vi "TLB Native Dynamic Events ver 0.26a.vi"() -> ()   [LabVIEW 2018] (continued)
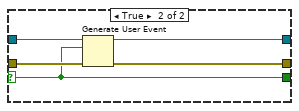
[diagram p2: hidden frame]
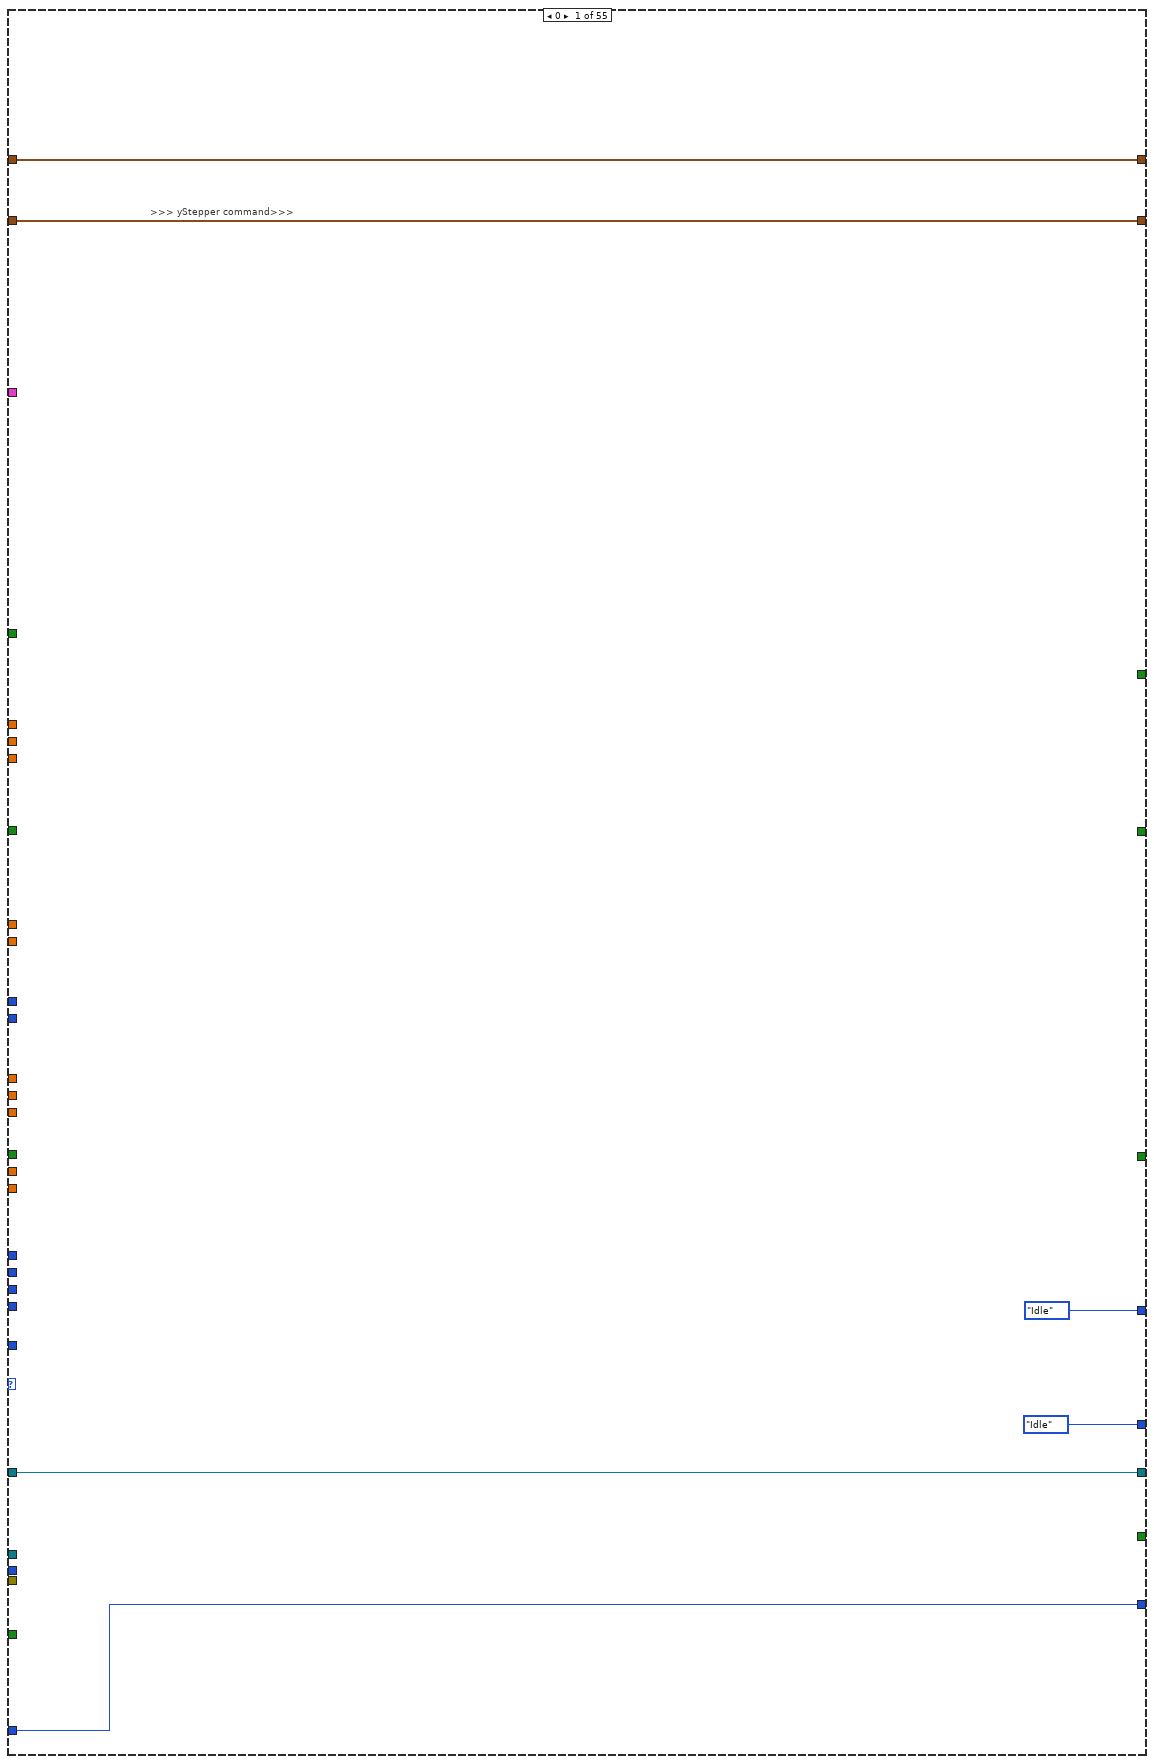
[diagram p5: hidden frame]
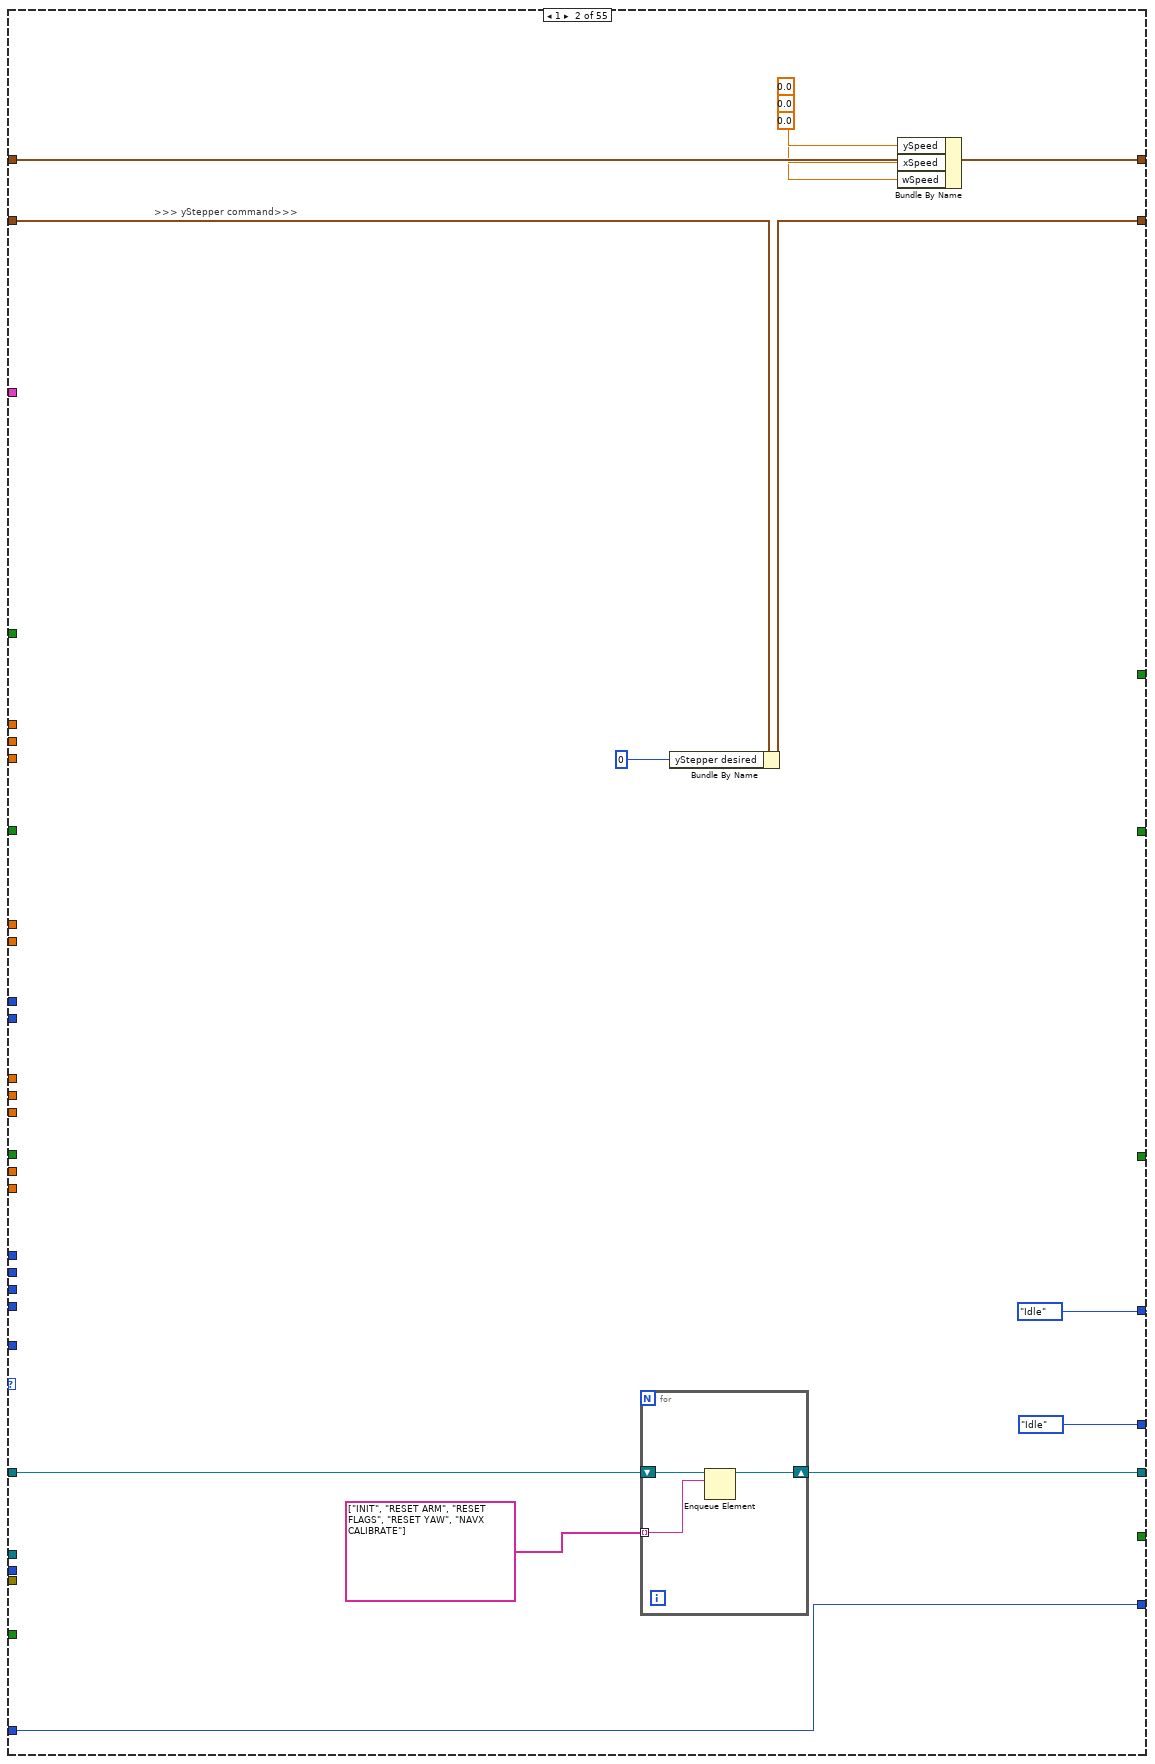
[diagram p6: hidden frame]
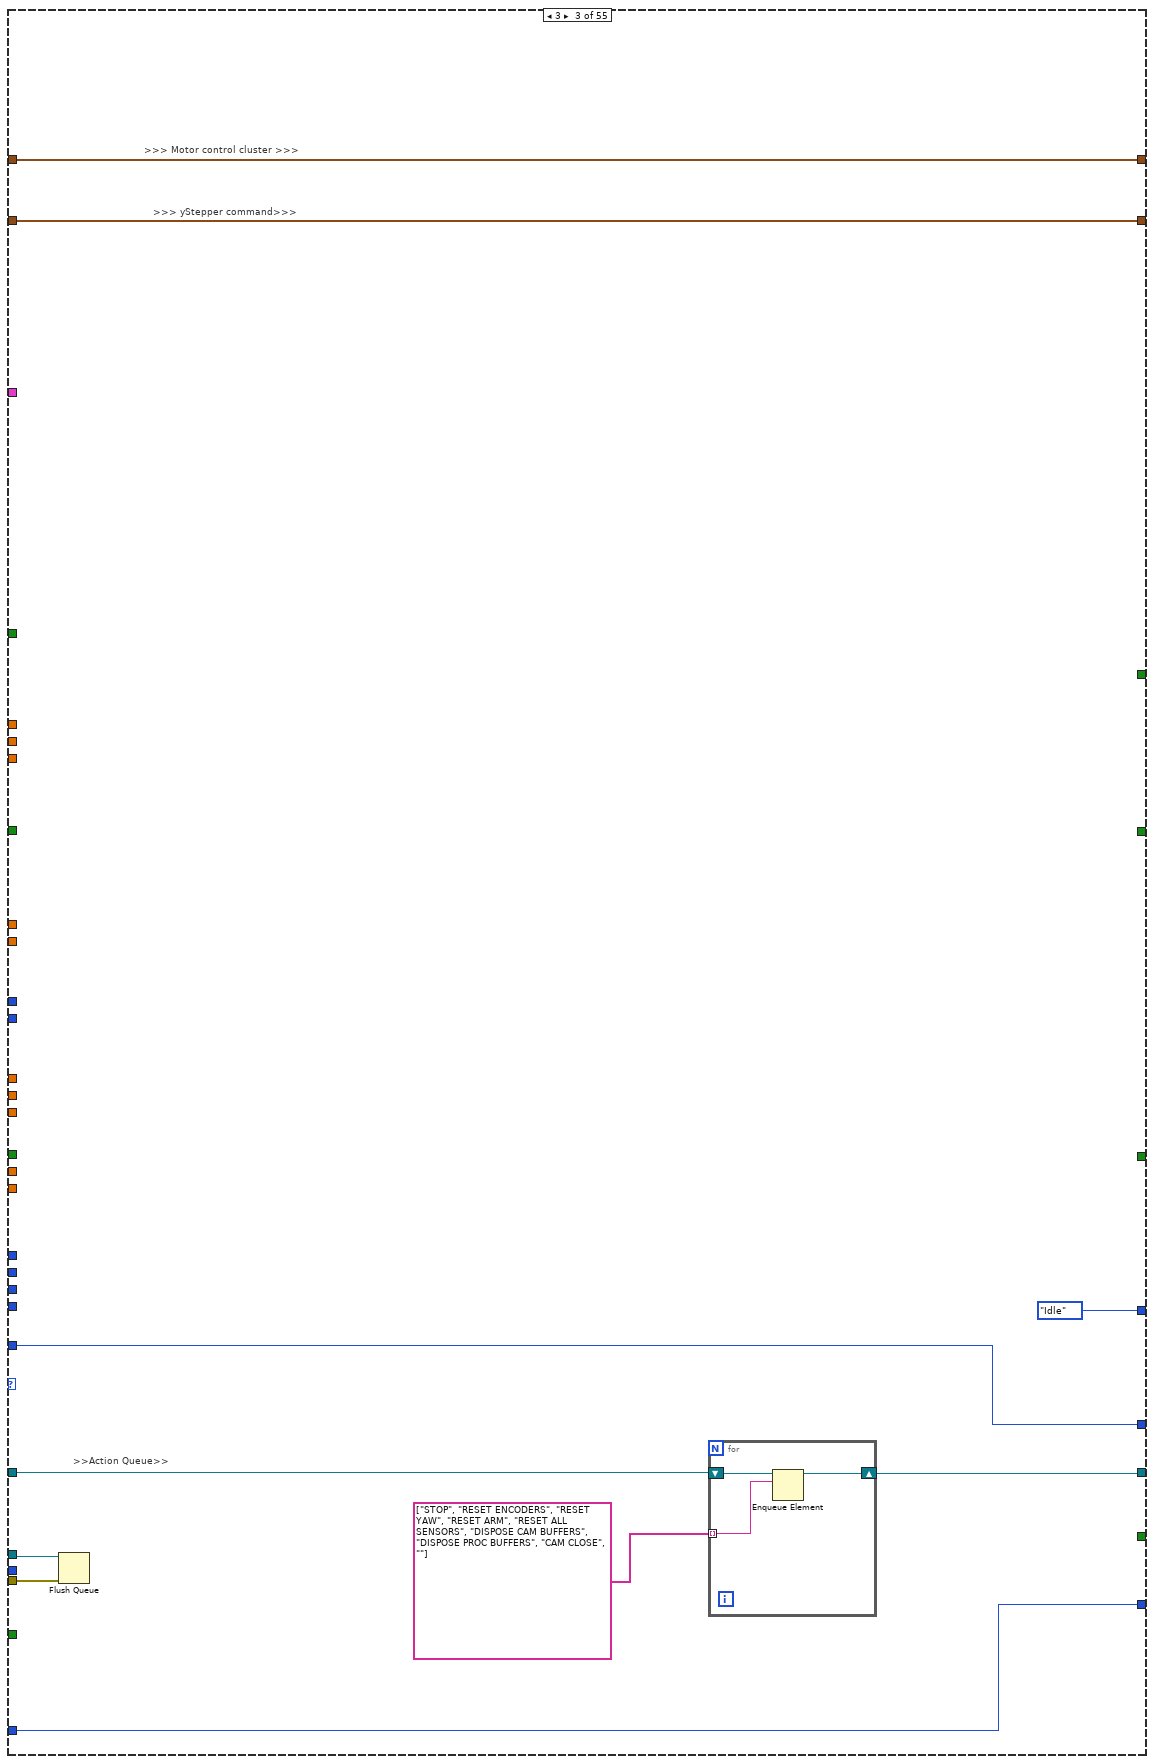
[diagram p7: hidden frame]
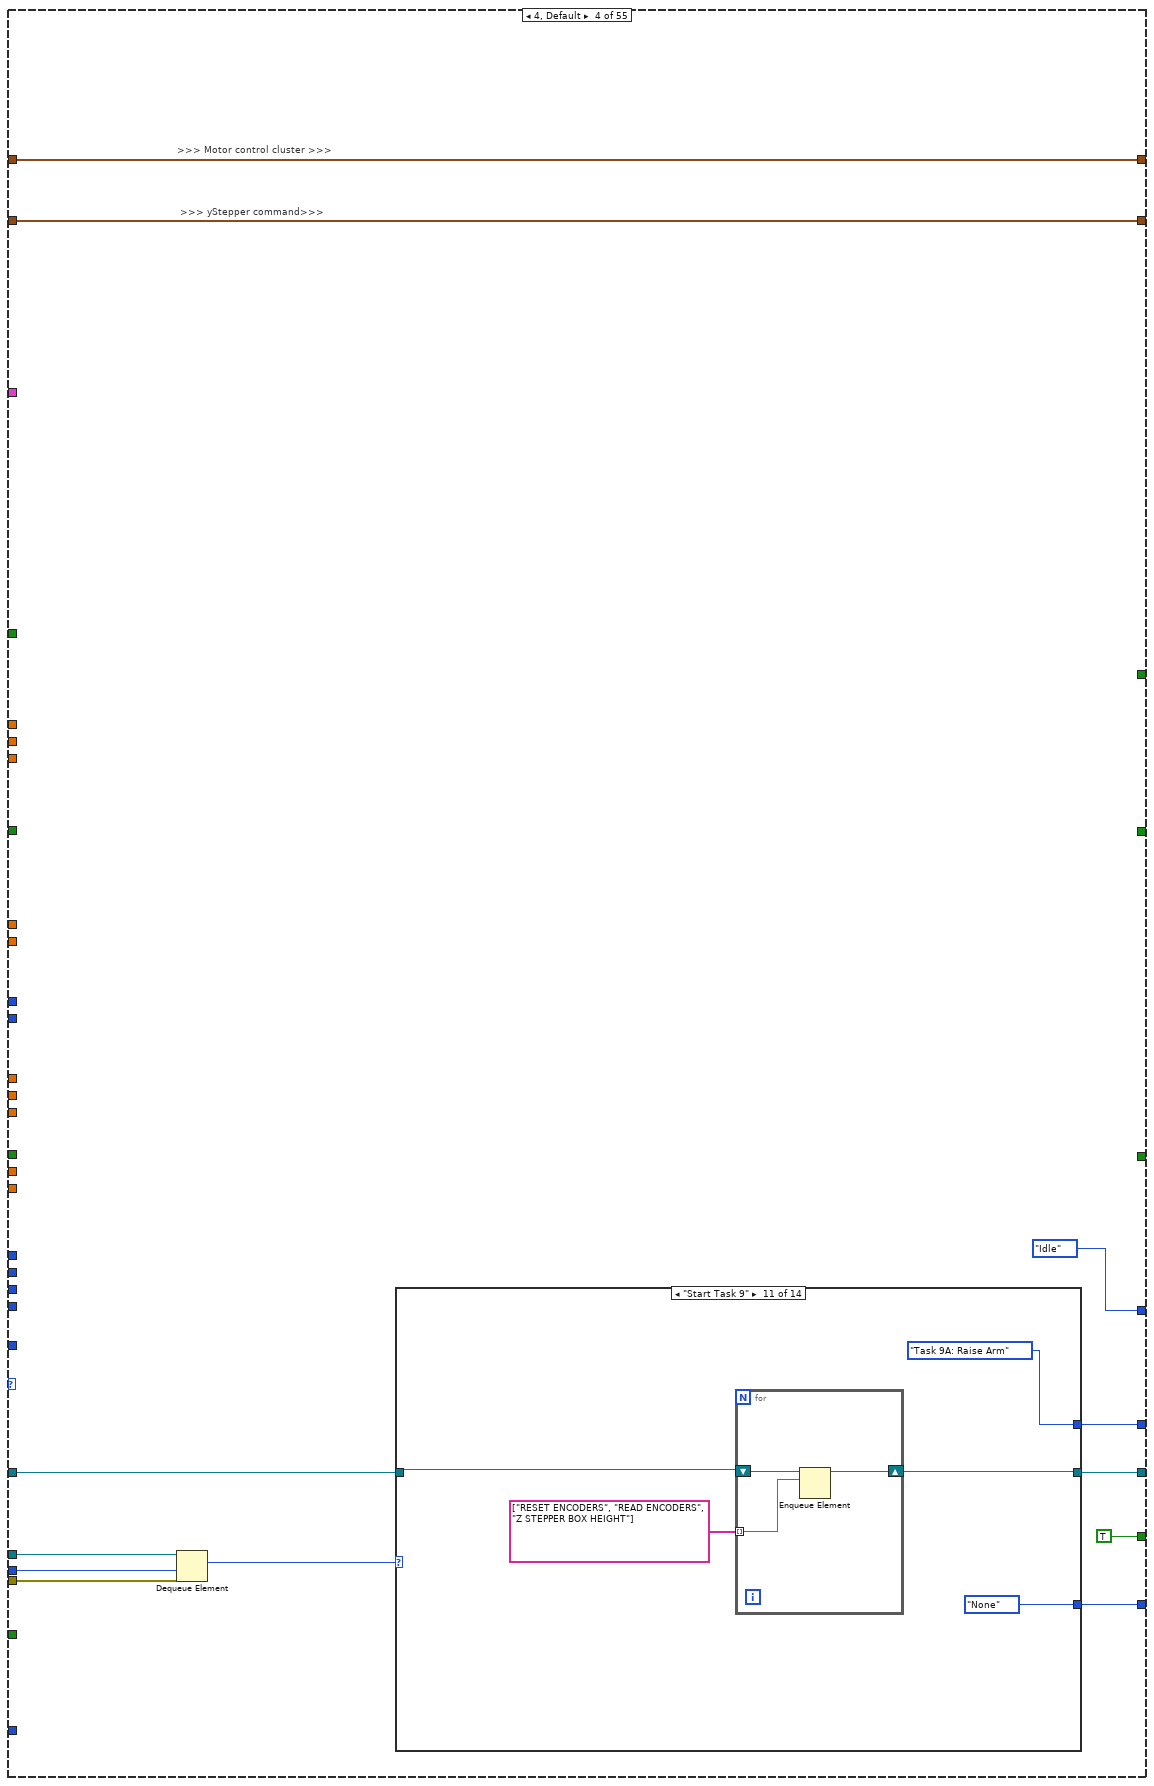
[diagram p8: hidden frame]
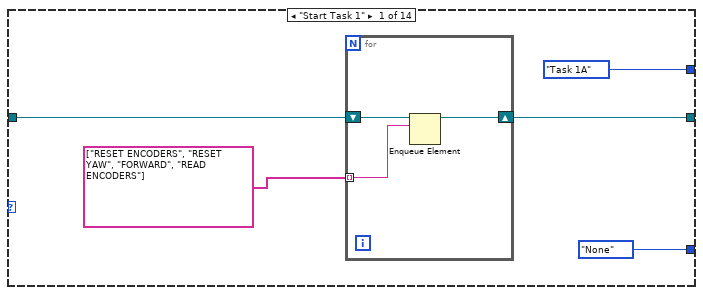
[diagram p9: hidden frame]
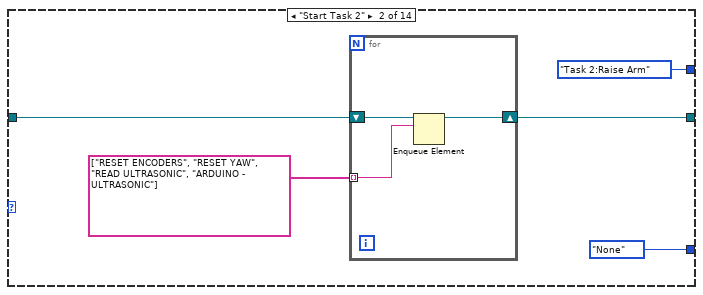
[diagram p10: hidden frame]
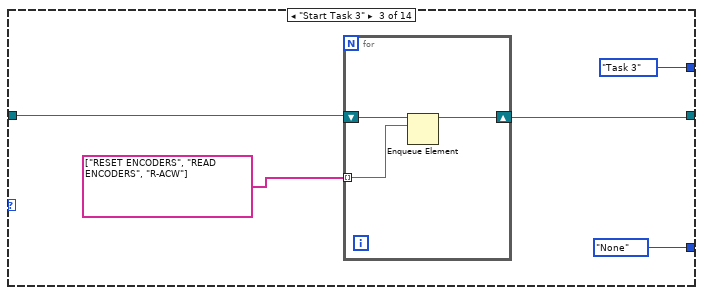
[diagram p11: hidden frame]
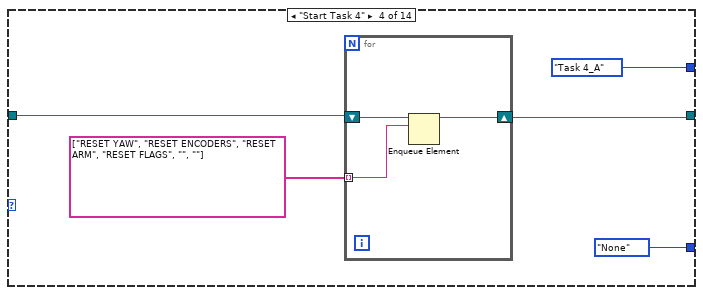
[diagram p12: hidden frame]
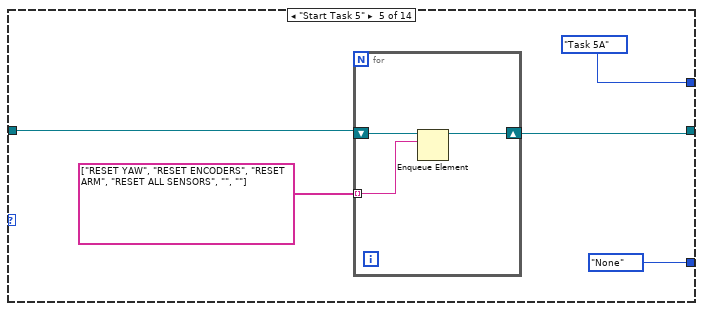
[diagram p13: hidden frame]
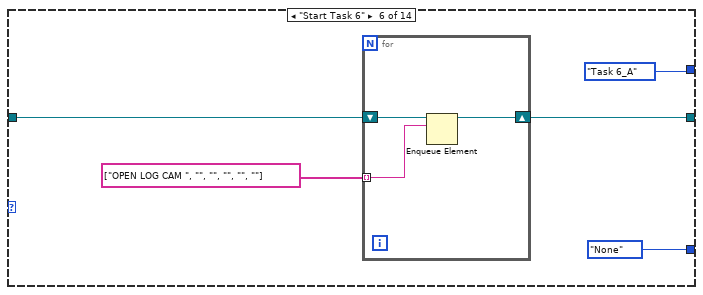
[diagram p14: hidden frame]
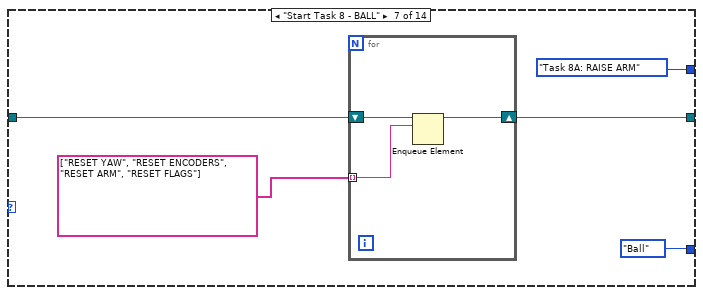
[diagram p15: hidden frame]
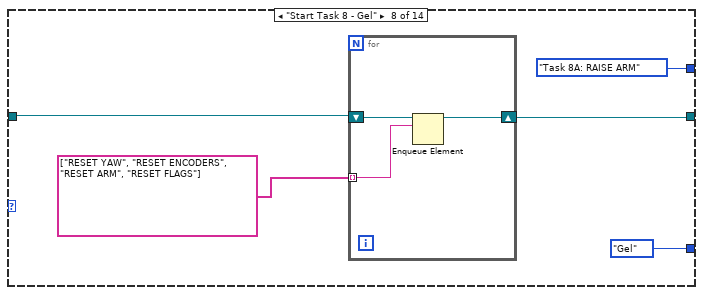
[diagram p16: hidden frame]
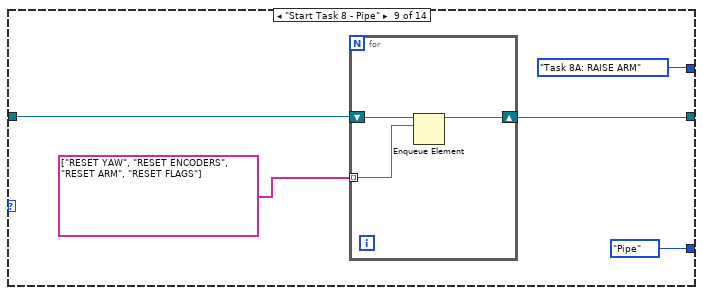
[diagram p17: hidden frame]
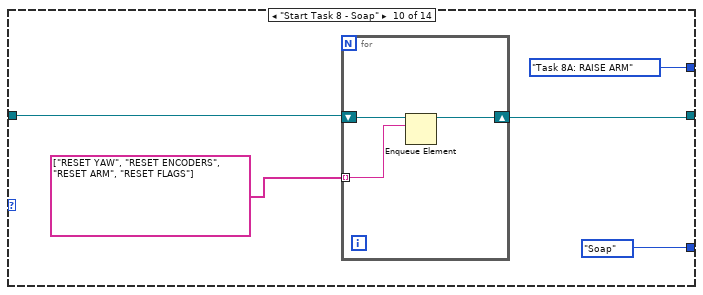
[diagram p18: hidden frame]
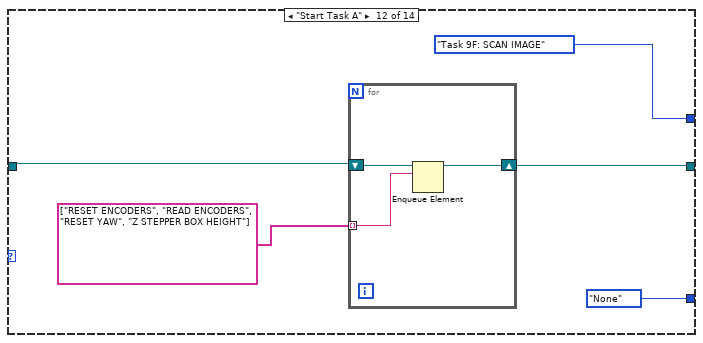
[diagram p19: hidden frame]
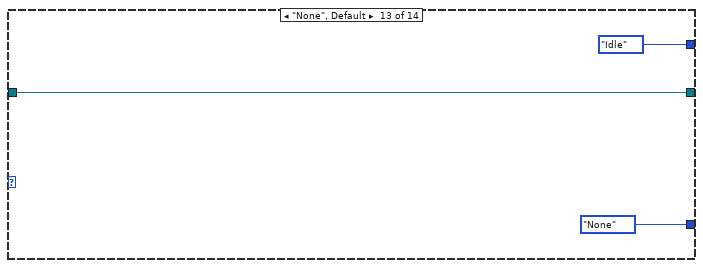
[diagram p20: hidden frame]
              frame "Start Task 1", Default {
                n815 = case shown="False" w2516 {
                  tunnel: w2522 -> [w2526 w2533]
                  tunnel: [w2527 w2532] -> w2521
                  frame False {
                    n816 = for {
                      tunnel: string[] ["READ LINE SENSOR", "READ NAVX", "RIGHT", "READ ENCODERS"] ("element") -> [w2528] mode=indexing
                      shift-right: [w2530] -> w2527
                      shift-left: w2526 -> [w2529]
                      n817 = Enqueue Element(queue=w2529, element=w2528) -> (queue out=w2530:refnum<queue>)  [unwired: 2 in, 2 out]
                    }
                  }
                  frame True {
                    n818 = for {
                      shift-right: [w2535] -> w2532
                      shift-left: w2533 -> [w2536]
                      tunnel: string[] ["STOP", "RESET ENCODERS", "RESET YAW", "OPEN LIFE CAM", "SET TIMER 2", "RESET FLAGS"] -> [w2534] mode=indexing
                      n819 = Enqueue Element(queue=w2536, element=w2534) -> (queue out=w2535:refnum<queue>)  [unwired: 2 in, 2 out]
                    }
                  }
                }
                n820 = Or(x=w2516, y=w2515) -> (x .or. y?=w2514:bool)
                n821 = Select(t=State_Type_Definitions,_for_0.26g_versions_and_later_2."True Stop" ("Enum"), s=w2515, f=State_Type_Definitions,_for_0.26d_versions_and_later."Task 9N: SCAN IMAGE" ("Enum")) -> (s? t:f=w2517:u16)
                n822 = Select(t=w2517, s=w2514, f=State_Type_Definitions,_for_0.26g_versions_and_later_2."Task 9M: MOVE RIGHT" ("Enum")) -> (s? t:f=w2523:u16)
              }
              frame "Exit" {
                n823 = for {
                  shift-right: [w2543] -> w2540
                  shift-left: w2539 -> [w2544]
                  tunnel: string[] ["STOP", "RESET ENCODERS", "RESET YAW", "ARDUINO MODE 0"] -> [w2542] mode=indexing
                  n824 = Enqueue Element(queue=w2544, element=w2542) -> (queue out=w2543:refnum<queue>)  [unwired: 2 in, 2 out]
                }
              }
            }
          }
          frame 51 {
            # ">> Manual override >>"
            n825 = Dequeue Element(queue=w2553, timeout in ms (-1)=w2552, error in (no error)=w2551) -> (element=w2554:T10)  [unwired: 3 out]
            n826 = case shown="\"Start Task 1\", Default" w2554 {
              tunnel: [w2568 State_Type_Definitions,_for_0.26g_versions_and_later_2."True Stop" ("Enum")] -> w2546
              tunnel: [w2566 w2584] -> w2545
              tunnel: w2549 -> [w2565 w2581]
              tunnel: w2550 -> [w2559 _]
              tunnel: [State_Type_Definitions,_for_0.26g_versions_and_later_2."Idle" ("Enum") State_Type_Definitions,_for_0.26g_versions_and_later_2."Shutdown" ("Enum")] -> w2547
              tunnel: w2548 -> [w2558 _]
              frame "Start Task 1", Default {
                # ">> WIill proceed to part ii if not manual override >>"
                # ">>If ENABLE or Trigger is set to true>>"
                n827 = Or(x=w2558, y=w2559) -> (x .or. y?=w2560:bool)
                n828 = case shown="False" w2558 {
                  tunnel: [w2571 w2577] -> w2566
                  tunnel: w2565 -> [w2570 w2576]
                  frame False {
                    n829 = for {
                      shift-right: [w2573] -> w2571
                      shift-left: w2570 -> [w2574]
                      tunnel: string[] ["CAM ACQ", "START TIMER"] ("element") -> [w2572] mode=indexing
                      n830 = Enqueue Element(queue=w2574, element=w2572) -> (queue out=w2573:refnum<queue>)  [unwired: 2 in, 2 out]
                    }
                  }
                  frame True {
                    n831 = for {
                      shift-right: [w2579] -> w2577
                      shift-left: w2576 -> [w2580]
                      tunnel: string[] ["CLOSE CAM", "SET TIMER 5", "", "", "", ""] -> [w2578] mode=indexing
                      n832 = Enqueue Element(queue=w2580, element=w2578) -> (queue out=w2579:refnum<queue>)  [unwired: 2 in, 2 out]
                    }
                  }
                }
                n833 = Select(t=State_Type_Definitions,_for_0.26g_versions_and_later_2."True Stop" ("Enum"), s=w2559, f=State_Type_Definitions,_for_0.26d_versions_and_later."Task 9O: PROCESS COLOUR" ("Enum")) -> (s? t:f=w2562:u16)
                n834 = Select(t=w2562, s=w2560, f=State_Type_Definitions,_for_0.26d_versions_and_later."Task 9N: SCAN IMAGE" ("Enum")) -> (s? t:f=w2568:u16)
              }
              frame "Exit" {
                n835 = for {
                  shift-right: [w2587] -> w2584
                  shift-left: w2581 -> [w2588]
                  tunnel: string[] ["STOP", "RESET ENCODERS", "RESET YAW", ""] -> [w2586] mode=indexing
                  n836 = Enqueue Element(queue=w2588, element=w2586) -> (queue out=w2587:refnum<queue>)  [unwired: 2 in, 2 out]
                }
              }
            }
          }
          frame 52 {
            # ">> Item Selection Bias >>"
            n837 = Dequeue Element(queue=w2596, timeout in ms (-1)=w2595, error in (no error)=w2594) -> (element=w2598:T10)  [unwired: 3 out]
            n838 = case shown="\"Start Task 1\", Default" w2598 {
              tunnel: w2589 -> [w2604 _]
              tunnel: [w2611 State_Type_Definitions,_for_0.26g_versions_and_later_2."True Stop" ("Enum")] -> w2592
              tunnel: w2593 -> [w2603 _]
              tunnel: w2597 -> [w2610 w2627]
              tunnel: [w2609 w2628] -> w2591
              tunnel: [State_Type_Definitions,_for_0.26g_versions_and_later_2."Idle" ("Enum") State_Type_Definitions,_for_0.26g_versions_and_later_2."Shutdown" ("Enum")] -> w2590
              frame "Start Task 1", Default {
                n839 = case shown="False" w2604 {
                  tunnel: w2610 -> [w2614 w2621]
                  tunnel: [w2615 w2620] -> w2609
                  frame False {
                    n840 = for {
                      tunnel: string[] ["START TIMER", "COLOUR PROCESSING", ""] ("element") -> [w2616] mode=indexing
                      shift-right: [w2618] -> w2615
                      shift-left: w2614 -> [w2617]
                      n841 = Enqueue Element(queue=w2617, element=w2616) -> (queue out=w2618:refnum<queue>)  [unwired: 2 in, 2 out]
                    }
                  }
                  frame True {
                    n842 = for {
                      shift-right: [w2623] -> w2620
                      shift-left: w2621 -> [w2624]
                      tunnel: string[] ["CLOSE CAM", "DISPOSE BUFFERS", "RESET ENCODERS", "RESET YAW", "RESET FLAGS", ""] -> [w2622] mode=indexing
                      n843 = Enqueue Element(queue=w2624, element=w2622) -> (queue out=w2623:refnum<queue>)  [unwired: 2 in, 2 out]
                    }
                  }
                }
                n844 = Or(x=w2604, y=w2603) -> (x .or. y?=w2602:bool)
                n845 = Select(t=State_Type_Definitions,_for_0.26g_versions_and_later_2."True Stop" ("Enum"), s=w2603, f=State_Type_Definitions,_for_0.26d_versions_and_later."Task 9P: MOVE RIGHT" ("Enum")) -> (s? t:f=w2605:u16)
                n846 = Select(t=w2605, s=w2602, f=State_Type_Definitions,_for_0.26d_versions_and_later."Task 9O: PROCESS COLOUR" ("Enum")) -> (s? t:f=w2611:u16)
              }
              frame "Exit" {
                n847 = for {
                  shift-right: [w2631] -> w2628
                  shift-left: w2627 -> [w2632]
                  tunnel: string[] ["STOP", "RESET ENCODERS", "RESET YAW", "ARDUINO MODE 0"] -> [w2630] mode=indexing
                  n848 = Enqueue Element(queue=w2632, element=w2630) -> (queue out=w2631:refnum<queue>)  [unwired: 2 in, 2 out]
                }
              }
            }
          }
          frame 53 {
            # ">> Item Selection Bias >>"
            n849 = Dequeue Element(queue=w2638, timeout in ms (-1)=w2637, error in (no error)=w2636) -> (element=w2646:T10)  [unwired: 3 out]
            n850 = Greater?(x=w2634, y=50.0) -> (0:w2644:bool)
            n851 = And(x=w2633, y=w2644) -> (x .and. y?=w2645:bool)
            n852 = case shown="\"Start Task 1\", Default" w2646 {
              tunnel: w2645 -> [w2652 _]
              tunnel: [w2659 State_Type_Definitions,_for_0.26g_versions_and_later_2."True Stop" ("Enum")] -> w2641
              tunnel: w2635 -> [w2651 _]
              tunnel: w2639 -> [w2658 w2675]
              tunnel: [w2657 w2676] -> w2640
              tunnel: [State_Type_Definitions,_for_0.26g_versions_and_later_2."Idle" ("Enum") State_Type_Definitions,_for_0.26g_versions_and_later_2."Shutdown" ("Enum")] -> w2642
              frame "Start Task 1", Default {
                n853 = case shown="False" w2652 {
                  tunnel: w2658 -> [w2662 w2669]
                  tunnel: [w2663 w2668] -> w2657
                  frame False {
                    n854 = for {
                      tunnel: string[] ["READ LINE SENSOR", "READ NAVX", "RIGHT", "READ ENCODERS"] ("element") -> [w2664] mode=indexing
                      shift-right: [w2666] -> w2663
                      shift-left: w2662 -> [w2665]
                      n855 = Enqueue Element(queue=w2665, element=w2664) -> (queue out=w2666:refnum<queue>)  [unwired: 2 in, 2 out]
                    }
                  }
                  frame True {
                    n856 = for {
                      shift-right: [w2671] -> w2668
                      shift-left: w2669 -> [w2672]
                      tunnel: string[] ["STOP", "RESET ENCODERS", "RESET YAW", "OPEN LIFE CAM", "SET TIMER 2", "RESET FLAGS"] -> [w2670] mode=indexing
                      n857 = Enqueue Element(queue=w2672, element=w2670) -> (queue out=w2671:refnum<queue>)  [unwired: 2 in, 2 out]
                    }
                  }
                }
                n858 = Or(x=w2652, y=w2651) -> (x .or. y?=w2650:bool)
                n859 = Select(t=State_Type_Definitions,_for_0.26g_versions_and_later_2."True Stop" ("Enum"), s=w2651, f=State_Type_Definitions,_for_0.26d_versions_and_later."Task 9Q: SCAN IMAGE" ("Enum")) -> (s? t:f=w2653:u16)
                n860 = Select(t=w2653, s=w2650, f=State_Type_Definitions,_for_0.26d_versions_and_later."Task 9P: MOVE RIGHT" ("Enum")) -> (s? t:f=w2659:u16)
              }
              frame "Exit" {
                n861 = for {
                  shift-right: [w2679] -> w2676
                  shift-left: w2675 -> [w2680]
                  tunnel: string[] ["STOP", "RESET ENCODERS", "RESET YAW", "ARDUINO MODE 0"] -> [w2678] mode=indexing
                  n862 = Enqueue Element(queue=w2680, element=w2678) -> (queue out=w2679:refnum<queue>)  [unwired: 2 in, 2 out]
                }
              }
            }
          }
          frame 54 {
            # ">> Manual override >>"
            n863 = Dequeue Element(queue=w2689, timeout in ms (-1)=w2688, error in (no error)=w2687) -> (element=w2690:T10)  [unwired: 3 out]
            n864 = case shown="\"Start Task 1\", Default" w2690 {
              tunnel: [w2704 State_Type_Definitions,_for_0.26g_versions_and_later_2."True Stop" ("Enum")] -> w2682
              tunnel: [w2702 w2720] -> w2681
              tunnel: w2685 -> [w2701 w2717]
              tunnel: w2686 -> [w2695 _]
              tunnel: [State_Type_Definitions,_for_0.26g_versions_and_later_2."Idle" ("Enum") State_Type_Definitions,_for_0.26g_versions_and_later_2."Shutdown" ("Enum")] -> w2683
              tunnel: w2684 -> [w2694 _]
              frame "Start Task 1", Default {
                # ">> WIill proceed to part ii if not manual override >>"
                # ">>If ENABLE or Trigger is set to true>>"
                n865 = Or(x=w2694, y=w2695) -> (x .or. y?=w2696:bool)
                n866 = case shown="False" w2694 {
                  tunnel: [w2707 w2713] -> w2702
                  tunnel: w2701 -> [w2706 w2712]
                  frame False {
                    n867 = for {
                      shift-right: [w2709] -> w2707
                      shift-left: w2706 -> [w2710]
                      tunnel: string[] ["CAM ACQ", "START TIMER"] ("element") -> [w2708] mode=indexing
                      n868 = Enqueue Element(queue=w2710, element=w2708) -> (queue out=w2709:refnum<queue>)  [unwired: 2 in, 2 out]
                    }
                  }
                  frame True {
                    n869 = for {
                      shift-right: [w2715] -> w2713
                      shift-left: w2712 -> [w2716]
                      tunnel: string[] ["CLOSE CAM", "SET TIMER 5", "", "", "", ""] -> [w2714] mode=indexing
                      n870 = Enqueue Element(queue=w2716, element=w2714) -> (queue out=w2715:refnum<queue>)  [unwired: 2 in, 2 out]
                    }
                  }
                }
                n871 = Select(t=State_Type_Definitions,_for_0.26g_versions_and_later_2."True Stop" ("Enum"), s=w2695, f=State_Type_Definitions,_for_0.26g_versions_and_later_2."Task 9R: PROCESS COLOUR" ("Enum")) -> (s? t:f=w2698:T18)
                n872 = Select(t=w2698, s=w2696, f=State_Type_Definitions,_for_0.26d_versions_and_later."Task 9Q: SCAN IMAGE" ("Enum")) -> (s? t:f=w2704:u16)
              }
              frame "Exit" {
                n873 = for {
                  shift-right: [w2723] -> w2720
                  shift-left: w2717 -> [w2724]
                  tunnel: string[] ["STOP", "RESET ENCODERS", "RESET YAW", ""] -> [w2722] mode=indexing
                  n874 = Enqueue Element(queue=w2724, element=w2722) -> (queue out=w2723:refnum<queue>)  [unwired: 2 in, 2 out]
                }
              }
            }
          }
          frame 55 {
            # ">> Item Selection Bias >>"
            # ">>> Motor control cluster >>>"
            # ">>> yStepper command>>>"
            n875 = Dequeue Element(queue=w2730, timeout in ms (-1)=w2731, error in (no error)=w2732) -> (element=w2734:T10)  [unwired: 3 out]
            n876 = case shown="\"Start Task 1\", Default" w2734 {
              tunnel: w2728 -> [w2740 _]
              tunnel: [w2747 State_Type_Definitions,_for_0.26g_versions_and_later_2."True Stop" ("Enum")] -> w2726
              tunnel: w2733 -> [w2739 _]
              tunnel: w2729 -> [w2746 w2763]
              tunnel: [w2745 w2764] -> w2725
              tunnel: [State_Type_Definitions,_for_0.26g_versions_and_later_2."Idle" ("Enum") State_Type_Definitions,_for_0.26g_versions_and_later_2."Shutdown" ("Enum")] -> w2727
              frame "Start Task 1", Default {
                n877 = case shown="False" w2740 {
                  tunnel: w2746 -> [w2750 w2757]
                  tunnel: [w2751 w2756] -> w2745
                  frame False {
                    n878 = for {
                      tunnel: string[] ["START TIMER", "COLOUR PROCESSING", ""] ("element") -> [w2752] mode=indexing
                      shift-right: [w2754] -> w2751
                      shift-left: w2750 -> [w2753]
                      n879 = Enqueue Element(queue=w2753, element=w2752) -> (queue out=w2754:refnum<queue>)  [unwired: 2 in, 2 out]
                    }
                  }
                  frame True {
                    n880 = for {
                      shift-right: [w2759] -> w2756
                      shift-left: w2757 -> [w2760]
                      tunnel: string[] ["CLOSE CAM", "DISPOSE BUFFERS", "RESET ENCODERS", "RESET YAW", "RESET FLAGS", ""] -> [w2758] mode=indexing
                      n881 = Enqueue Element(queue=w2760, element=w2758) -> (queue out=w2759:refnum<queue>)  [unwired: 2 in, 2 out]
                    }
                  }
                }
                n882 = Or(x=w2740, y=w2739) -> (x .or. y?=w2738:bool)
                n883 = Select(t=State_Type_Definitions,_for_0.26g_versions_and_later_2."True Stop" ("Enum"), s=w2739, f=State_Type_Definitions,_for_0.26g_versions_and_later_2."True Stop" ("Enum")) -> (s? t:f=w2741:T18)
                n884 = Select(t=w2741, s=w2738, f=State_Type_Definitions,_for_0.26g_versions_and_later_2."Task 9R: PROCESS COLOUR" ("Enum")) -> (s? t:f=w2747:T18)
              }
              frame "Exit" {
                n885 = for {
                  shift-right: [w2767] -> w2764
                  shift-left: w2763 -> [w2768]
                  tunnel: string[] ["STOP", "RESET ENCODERS", "RESET YAW", "ARDUINO MODE 0"] -> [w2766] mode=indexing
                  n886 = Enqueue Element(queue=w2768, element=w2766) -> (queue out=w2767:refnum<queue>)  [unwired: 2 in, 2 out]
                }
              }
            }
          }
        }
        "Object Detection" <- w313
        "Ultrasonic sensors" <- w336
        "Encoder values" <- w325
        "Stepper position values" <- w309
        "NAVX Values" <- w307
        "IR Sensors" <- w299
        "Line sensors" <- w294
        "Time cluster" <- w305
        "Box Colour Detection" <- w287
      }
    }
    "Object recognition mode" <- w220
    "Front Ultrasonic obstruct" <- w217
    "Front IR obstruct" <- w216
    "Table IR obstruct" <- w215
    n887 = local write "Green LED"(w230) -> ()
  }
  n888 = while {
    stop <- w3609 stop-if-true
    n889 = call "MOTOR CONTROL WITH PID AE.vi"("AE Mode"=MOTOR_CONTROL_WITH_PID_AE_DATA_MODE_TYPE_DEF."Read from AE") -> ("Speed & distance"=→"Speed & distance":T15)  [unwired: 3 in]
    n890 = call "FGV Stop.vi"("Init/Read/Write State"=States_for_Action_Engine."Read") -> ("Output node"=w3609:bool)  [unwired: 2 in, 1 out]
    n891 = Wait (ms)(milliseconds to wait=u32 5) -> ()  [unwired: 1 out]
  }
  n892 = call <vilib>:"DIO Close.vi"("error in (no error)"=w23, "DIO Info In"=w26) -> ()  [unwired: 9 in, 1 out]
  n893 = call <vilib>:"DIO Close.vi"("error in (no error)"=w33, "DIO Info In"=w35) -> ()  [unwired: 9 in, 1 out]
  n894 = call <vilib>:"NavX Close.vi"("error in (no error)"=w10, "NavX Info In"=w9) -> ()  [unwired: 9 in, 1 out]
  n895 = call <vilib>:"DIO Close.vi"("error in (no error)"=w28, "DIO Info In"=w30) -> ()  [unwired: 9 in, 1 out]
  n896 = call <vilib>:"DIO Close.vi"("error in (no error)"=w17, "DIO Info In"=w18) -> ()  [unwired: 9 in, 1 out]
  n897 = call <vilib>:"DIO Close.vi"("error in (no error)"=w12, "DIO Info In"=w13) -> ()  [unwired: 9 in, 1 out]
  n898 = Merge Errors "Merge Errors"(w63, w62) -> (w45:errorcluster)
  n899 = Merge Errors(w49, w45) -> (w44:errorcluster)
  n900 = Destroy User Event(user event=w67, error in=w44) -> ()  [unwired: 1 out]
  n901 = Release Queue(queue=w40, error in (no error)=w44) -> (error out=→"Queue Errors":errorcluster)  [unwired: 1 in, 2 out]
  n902 = Release Queue(queue=w57, error in (no error)=w44) -> ()  [unwired: 1 in, 3 out]
  n903 = Destroy User Event(user event=w66, error in=w44) -> ()  [unwired: 1 out]
  n904 = Unregister For Events(event registration refnum=w58, error in=w44) -> ()  [unwired: 1 out]
